vi "UHR-Fleezers Control (host) - 12.2.vi"() -> ()   [LabVIEW 2014] (continued)
                                n838 = flat-sequence {
                                tunnel: [w1198] -> w1193
                                tunnel: w1192 -> [w1198]
                                tunnel: [w1194] -> w1191
                                tunnel: w1190 -> [w1194]
                                tunnel: w1193 -> [w1201]
                                tunnel: w1191 -> [w1199]
                                frame #0 {
                                n839 = local read "Yank Delay (s)"() -> (w1197:dbl)
                                n840 = Multiply(x=w1197, y=1000.0) -> (x*y=w1195:dbl)
                                n841 = Wait (ms)(milliseconds to wait=w1195) -> ()  [unwired: 1 out]
                                }
                                frame #1 {
                                n842 = local read "Yank to which?"() -> (w1200:bool)
                                n843 = case shown="False" w1200 {
                                tunnel: w1201 -> [_ w1229]
                                tunnel: w1199 -> [w1202 _]
                                frame False {
                                n844 = flat-sequence {
                                tunnel: w1202 -> [w1203]
                                frame #0 {
                                n845 = property on="Trap Pos FB SP" class="DigNum (strict)"("Val(Sgnl)"=w1203) -> ()  [unwired: 2 in, 2 out]
                                }
                                frame #1 {
                                n846 = Wait (ms)(milliseconds to wait=u32 700) -> ()  [unwired: 1 out]
                                }
                                frame #2 {
                                n847 = local read "Action (%)"() -> (w1208:dbl)
                                n848 = Absolute Value(x=w1208) -> (abs(x)=w1207:dbl)
                                n849 = Greater?(x=w1207, y=70.0) -> (0:w1205:bool)
                                n850 = property on="Remove Action Offset" class="Bool (strict)"("Val(Sgnl)"=w1205) -> ()  [unwired: 2 in, 2 out]
                                }
                                frame #3 {
                                n851 = for {
                                N: 4 -> [_]
                                n852 = flat-sequence {
                                frame #0 {
                                n853 = Wait (ms)(milliseconds to wait=u32 500) -> ()  [unwired: 1 out]
                                }
                                frame #1 {
                                n854 = local read "Action (%)"() -> (w1214:dbl)
                                n855 = Absolute Value(x=w1214) -> (abs(x)=w1213:dbl)
                                n856 = Greater?(x=w1213, y=70.0) -> (0:w1211:bool)
                                n857 = property on="Remove Action Offset" class="Bool (strict)"("Val(Sgnl)"=w1211) -> ()  [unwired: 2 in, 2 out]
                                }
                                }
                                }
                                }
                                frame #4 {
                                n858 = local read "Shift confocal"() -> (w1219:bool)
                                n859 = local read "Mean"() -> (w1221:dbl)
                                n860 = Greater?(x=w1221, y=11.0) -> (0:w1218:bool)
                                n861 = Not(x=w1218) -> (.not. x?=w1217:bool)
                                n862 = And(x=w1218, y=w1219) -> (x .and. y?=w1216:bool)
                                n863 = And(x=w1217, y=w1219) -> (x .and. y?=w1215:bool)
                                n864 = case shown="True" w1216 {
                                frame False {
                                }
                                frame True {
                                n865 = local read "Confocal Y 2 (V)"() -> (w1225:dbl)
                                n866 = local read "Confocal X 2 (V)"() -> (w1224:dbl)
                                n867 = property on="AO2" class="Slide (strict)"("Val(Sgnl)"=w1224) -> ()  [unwired: 2 in, 2 out]
                                n868 = property on="AO1" class="Slide (strict)"("Val(Sgnl)"=w1225) -> ()  [unwired: 2 in, 2 out]
                                }
                                }
                                n869 = case shown="True" w1215 {
                                frame False {
                                }
                                frame True {
                                n870 = local read "Confocal X 1 (V)"() -> (w1222:dbl)
                                n871 = local read "Confocal Y 1 (V)"() -> (w1223:dbl)
                                n872 = property on="AO1" class="Slide (strict)"("Val(Sgnl)"=w1223) -> ()  [unwired: 2 in, 2 out]
                                n873 = property on="AO2" class="Slide (strict)"("Val(Sgnl)"=w1222) -> ()  [unwired: 2 in, 2 out]
                                }
                                }
                                }
                                frame #5 {
                                n874 = Wait (ms)(milliseconds to wait=u32 1500) -> ()  [unwired: 1 out]
                                }
                                frame #6 {
                                n875 = property on="Rem fb disp offset" class="Bool (strict)"("Val(Sgnl)"=TRUE ("Value (Signaling)")) -> ()  [unwired: 2 in, 2 out]
                                n876 = property on="Remove Offset" class="Bool (strict)"("Val(Sgnl)"=TRUE ("Value (Signaling)")) -> ()  [unwired: 2 in, 2 out]
                                }
                                }
                                }
                                frame True {
                                n877 = flat-sequence {
                                tunnel: w1229 -> [w1230]
                                frame #0 {
                                n878 = property on="Trap D (MHz)" class="DigNum (strict)"("Val(Sgnl)"=w1230) -> ()  [unwired: 2 in, 2 out]
                                }
                                frame #1 {
                                n879 = Wait (ms)(milliseconds to wait=u32 500) -> ()  [unwired: 1 out]
                                }
                                frame #2 {
                                n880 = local read "Shift confocal"() -> (w1236:bool)
                                n881 = local read "Mean"() -> (w1238:dbl)
                                n882 = Greater?(x=w1238, y=11.0) -> (0:w1235:bool)
                                n883 = Not(x=w1235) -> (.not. x?=w1234:bool)
                                n884 = And(x=w1235, y=w1236) -> (x .and. y?=w1233:bool)
                                n885 = And(x=w1234, y=w1236) -> (x .and. y?=w1232:bool)
                                n886 = case shown="True" w1233 {
                                frame False {
                                }
                                frame True {
                                n887 = local read "Confocal Y 2 (V)"() -> (w1242:dbl)
                                n888 = local read "Confocal X 2 (V)"() -> (w1241:dbl)
                                n889 = property on="AO2" class="Slide (strict)"("Val(Sgnl)"=w1241) -> ()  [unwired: 2 in, 2 out]
                                n890 = property on="AO1" class="Slide (strict)"("Val(Sgnl)"=w1242) -> ()  [unwired: 2 in, 2 out]
                                }
                                }
                                n891 = case shown="True" w1232 {
                                frame False {
                                }
                                frame True {
                                n892 = local read "Confocal Y 1 (V)"() -> (w1240:dbl)
                                n893 = local read "Confocal X 1 (V)"() -> (w1239:dbl)
                                n894 = property on="AO2" class="Slide (strict)"("Val(Sgnl)"=w1239) -> ()  [unwired: 2 in, 2 out]
                                n895 = property on="AO1" class="Slide (strict)"("Val(Sgnl)"=w1240) -> ()  [unwired: 2 in, 2 out]
                                }
                                }
                                }
                                }
                                }
                                }
                                }
                                }
                                }
                                }
                                n896 = local read "Messages"() -> (w1187:string)
                                n897 = Subtract(x=w1179, y=w1178) -> (x-y=w1185:dbl)
                                "Duration (s)" <- w1185
                                n898 = Number To Decimal String(number=w1185, width (-)=i16 0) -> (decimal integer string=w1183:string)
                                n899 = Concatenate Strings(w1183, " s fluorescence event." ("string")) -> (w1181:string)
                                n900 = call "Update messages.vi"("Message to add"=w1181, "Old message string"=w1187) -> ("New message string"=w1186:string)
                                n901 = local write "Reset Force"(FALSE ("Reset Force")) -> ()
                                n902 = local write "Waiting"(TRUE ("Waiting")) -> ()
                                n903 = local write "Messages"(w1186) -> ()
                                n904 = local write "Fl. High"(FALSE ("Fl. High")) -> ()
                                n905 = call <vilib>:"Beep.vi"() -> ()  [unwired: 3 in, 9 out]
                                }
                                }
                                n906 = node-c288() -> ()  [unwired: 2 out]
                              }
                              n907 = node-c288(w1155) -> ()  [unwired: 1 out]
                            }
                          }
                        }
                      }
                      n908 = local read "Trap Pos FB SP"() -> (w1063:fxp<+/-,16,1>)
                      n909 = local read "Trap D (MHz)"() -> (w1068:dbl)
                    }
                  }
                }
                frame #1 {
                  n910 = local read "Stop All"() -> (w1252:bool)
                  n911 = local read "Fl. Triggered..."() -> (w1250:bool)
                  n912 = Not(x=w1250) -> (.not. x?=w1251:bool)
                  n913 = Or(x=w1251, y=w1252) -> (x .or. y?=w1249:bool)
                }
              }
              n914 = case shown="True" w838 {
                frame False {
                }
                frame True {
                  n915 = local read "Confocal Y 1 (V)"() -> (w848:dbl)
                  n916 = local read "Confocal X 1 (V)"() -> (w847:dbl)
                  n917 = property on="AO2" class="Slide (strict)"("Val(Sgnl)"=w847) -> ()  [unwired: 2 in, 2 out]
                  n918 = property on="AO1" class="Slide (strict)"("Val(Sgnl)"=w848) -> ()  [unwired: 2 in, 2 out]
                }
              }
              n919 = case shown="True" w838 {
                frame False {
                }
                frame True {
                  w846 = FALSE ("Fl. High")
                  n920 = local write "Waiting"(w846) -> ()
                  n921 = local write "Fl. High"(w846) -> ()
                }
              }
              n922 = node-c288() -> ()  [unwired: 2 out]
            }
            n923 = node-c288(w836) -> ()  [unwired: 1 out]
          }
        }
      }
      event "Stop All": Value Change {
        n924 = event-data() -> ()  [unwired: 7 out]
        n925 = local read "Stop All"() -> (w1257:bool)
      }
    }
    n926 = node-c288() -> ()  [unwired: 2 out]
  }
  n927 = property on="Saved trap pos" class="WFGraph (strict)"("Visible"=TRUE) -> ()  [unwired: 2 in, 2 out]
  n928 = property on="Trap Delta Graph" class="WFGraph (strict)"("Visible"=FALSE) -> ()  [unwired: 2 in, 2 out]
  n929 = local write "Trap pos"(TRUE ("Trap pos")) -> ()
  n930 = node-c288(2 ("Processor")) -> (w137:T26)  [unwired: 3 out]
  n931 = timed-loop "Control parameters (event loop)" {
    tunnel: w51 -> [w1266]
    shift-right: [w1265] -> _
    shift-left: errorcluster {"status"=FALSE, "code"=0, "source"=""} ("error out") -> [w1264]
    tunnel: [w1263] -> _
    timing: w137 -> [_]
    timing-out: [_] -> w136
    tunnel: w111 -> [w1262]
    tunnel: w55 -> [w1261]
    tunnel: w54 -> [w1260]
    tunnel: w53 -> [w1259]
    tunnel: w52 -> [w1258]
    stop <- w1263 stop-if-true
    n932 = node-c288() -> ()  [unwired: 2 out]
    n933 = event shown="[0] \"AI Count (ticks)\", \"Sets to FIFO (Traps)\", \"Save ave N\", \"FPGA Ave.\", \"# Samples/channel\", \"N sets to save\": Value Change" {
      selector: _ -> [_ _ _ _ _ _ _ _ _ _ _ _ _ _ _ _ _ _ _ _ _ _ _ _ _ _ _ _ _ _ _ _ _ _ _ _ _ _ _ _ _ _ _ _ _ _ _ _ _ _ _ _ _ _ _ _ _ _ _ _ _ _ _ _ _ _ _ _ _ _ _ _ _ _ _ _ _ _ _ _]
      dyn-events: _ -> [_ _ _ _ _ _ _ _ _ _ _ _ _ _ _ _ _ _ _ _ _ _ _ _ _ _ _ _ _ _ _ _ _ _ _ _ _ _ _ _ _ _ _ _ _ _ _ _ _ _ _ _ _ _ _ _ _ _ _ _ _ _ _ _ _ _ _ _ _ _ _ _ _ _ _ _ _ _ _ _]
      timeout: _ -> [_ _ _ _ _ _ _ _ _ _ _ _ _ _ _ _ _ _ _ _ _ _ _ _ _ _ _ _ _ _ _ _ _ _ _ _ _ _ _ _ _ _ _ _ _ _ _ _ _ _ _ _ _ _ _ _ _ _ _ _ _ _ _ _ _ _ _ _ _ _ _ _ _ _ _ _ _ _ _ _]
      tunnel: w1266 -> [w1304 _ _ _ w1342 _ w1364 _ _ _ _ w1430 _ _ w1473 w1479 w1484 w1490 w1526 w1553 w1563 _ w1582 w1586 w1597 w1608 w1619 w1636 w1647 w1658 w1685 w1779 w1786 w1824 _ _ w1884 w1888 w1899 w1903 w1907 _ w1915 _ _ _ _ _ _ _ _ _ _ _ _ _ _ _ _ _ w2296 _ w2313 _ w2320 w2338 _ w2345 w2353 w2368 w2379 w2385 _ w2394 _ w2413 _ _ _ w2488]
      tunnel: [w1303 _ _ _ w1332 _ w1363 _ _ w1395 _ w1409 _ _ w1472 w1475 w1481 w1487 w1525 w1551 w1562 _ w1580 _ w1591 w1602 w1613 w1630 w1641 w1652 w1683 w1777 w1784 w1822 _ _ w1882 w1886 w1889 w1901 w1905 _ w1913 _ _ _ _ _ _ _ _ _ _ _ _ _ _ _ _ _ w2294 _ _ _ _ w2335 _ _ _ _ _ _ _ _ _ _ _ _ _ w2486] -> w1265
      tunnel: w1264 -> [w1302 _ _ _ w1341 _ w1362 _ _ w1395 _ w1429 _ _ w1471 w1474 w1480 w1486 w1524 w1552 w1561 _ w1581 w1585 w1596 w1607 w1618 w1635 w1646 w1657 w1684 w1778 w1785 w1823 _ _ w1883 w1887 w1898 w1902 w1906 _ w1914 _ _ _ _ _ _ _ _ _ _ _ _ _ _ _ _ _ w2295 _ w2312 _ w2319 w2337 _ w2344 w2352 w2367 w2378 w2384 _ w2393 _ w2412 _ _ _ w2487]
      tunnel: [_ _ _ _ _ _ _ _ _ w1394 _ _ _ _ _ _ _ _ _ _ _ _ _ _ _ _ _ _ _ _ _ _ _ _ _ _ _ _ _ _ _ _ _ _ _ _ _ _ _ _ _ _ _ _ _ _ _ _ _ _ _ _ _ _ _ _ _ _ _ _ _ _ _ _ _ _ _ _ _ _] -> w1263
      tunnel: [_ _ _ _ _ _ _ "Round T1 X" _ _ _ _ _ _ _ _ _ _ _ _ _ _ _ _ _ _ _ _ _ _ _ _ _ _ _ _ _ _ _ _ _ _ _ _ _ _ _ _ _ _ _ _ _ _ _ _ _ _ _ _ _ _ _ _ _ _ _ _ _ _ _ _ _ _ _ _ _ _ _ _] -> _
      tunnel: [_ _ _ "Adjust Scale\nto Mean" _ _ _ _ _ _ _ _ _ _ _ _ _ _ _ _ _ _ "Test ttrig" _ _ _ _ _ _ _ _ _ _ _ _ _ _ _ _ _ _ _ _ _ _ _ _ _ _ _ "Flush Sample" "Flush Pump 3" "Flush Pump 1" "Clear Volume" _ _ _ _ _ _ _ _ _ _ _ _ _ _ _ _ _ _ _ _ _ _ _ _ _ _] -> _
      tunnel: [_ _ _ _ _ _ _ _ "Round T2 X" _ "Delayed Interlace Start" _ _ _ _ _ _ _ _ _ _ _ _ _ _ _ _ _ _ _ _ _ _ _ _ _ _ _ _ _ _ _ _ _ _ _ _ _ _ _ _ _ _ _ _ _ _ _ _ _ _ _ _ _ _ _ _ _ _ _ _ _ _ _ _ _ _ _ _ _] -> _
      tunnel: w1262 -> [_ _ _ _ _ _ _ _ _ _ _ _ _ _ _ _ _ _ _ _ _ _ _ _ _ _ _ _ _ _ _ _ _ _ _ _ _ _ _ _ _ _ _ _ _ _ w2073 w2091 w2098 w2103 w2109 _ _ w2208 _ _ _ _ _ _ _ _ _ _ _ _ _ _ _ _ _ _ _ _ _ _ _ _ _ _]
      tunnel: w1261 -> [_ _ _ _ _ _ _ _ _ _ _ _ _ _ _ _ _ _ _ _ _ _ _ _ _ _ _ _ _ _ _ _ _ _ _ _ _ _ _ _ _ _ _ _ w1989 _ _ _ _ _ _ w2139 _ _ w2215 _ w2224 _ w2238 _ _ _ _ _ _ _ _ _ _ _ _ _ _ _ _ _ _ _ _ _]
      tunnel: w1260 -> [_ _ _ _ _ _ _ _ _ _ _ _ _ _ _ _ _ _ _ _ _ _ _ _ _ _ _ _ _ _ _ _ _ _ _ _ _ _ _ _ _ _ _ _ _ _ _ _ _ _ _ _ _ _ _ _ _ _ _ _ _ _ _ _ _ _ _ _ _ _ _ _ _ _ _ _ _ _ _ _]
      tunnel: w1259 -> [_ _ _ _ _ _ _ _ _ _ _ _ _ _ _ _ _ _ _ _ _ _ _ _ _ _ _ _ _ _ _ _ _ _ _ _ _ _ _ _ _ _ _ w1926 _ _ _ _ _ _ _ _ w2169 _ _ w2220 _ w2231 _ w2263 _ _ _ _ _ _ _ _ _ _ _ _ _ _ _ _ _ _ _ _]
      tunnel: w1258 -> [_ _ _ _ _ _ _ _ _ _ _ _ _ _ _ _ _ _ _ _ _ _ _ _ _ _ _ _ _ _ _ _ _ _ _ _ _ _ _ _ _ _ _ _ _ _ _ _ _ _ _ _ _ _ _ _ _ _ _ _ _ _ _ _ _ _ _ _ _ _ _ _ _ _ _ _ _ _ _ _]
      event "AI Count (ticks)", "Sets to FIFO (Traps)", "Save ave N", "FPGA Ave.", "# Samples/channel", "N sets to save": Value Change {
        # "So that if 'Save ave N' is updated, the AOD scanning code updates too."
        n934 = event-data() -> ()  [unwired: 6 out]
        n935 = local read "AI Count (ticks)"() -> (w1284:u32)
        n936 = Boolean To (0,1)(Boolean="Sets to FIFO (Traps)") -> (0, 1=w1294:cluster{"Set 1":i16, "Set 2":i16, "Set 3":i16})
        n937 = Cluster To Array(cluster=w1294) -> (array=w1293:i16[])
        n938 = xnode "Read/Write Control"("FPGA VI Reference In"=w1304, "error in"=w1302, "ai count"=w1284, "AI1 Sets to FIFO"="Sets to FIFO (Traps)", "N of AI1 Int Acq Sets"="N Acq Sets (Traps + Fl.)") -> ("error out"=w1303:errorcluster)  [unwired: 1 out]
        n939 = To Unsigned Long Integer(number=w1293) -> (unsigned 32bit integer=w1273:u32[])
        n940 = local read "Scan steps (AOD)"() -> (w1295:u64)
        n941 = Multiply(x=w1284, y="N Acq Sets (Traps + Fl.)") -> (x*y=w1282:u32)
        n942 = Divide(x=40000000.0, y=w1284) -> (x/y=w1276:dbl)
        "AI rate (Hz)" <- w1276
        "Ave. Rate (Hz)" <- w1276
        n943 = Add Array Elements(numeric array=w1273) -> (sum=w1285:u32)
        "Trap Sets" <- w1285
        n944 = Reciprocal(x=w1276) -> (1/x=→"Ave. Period (s)":dbl)
        n945 = property on="Scan steps (AOD)" class="DigNum (strict)"("Val(Sgnl)"=w1295) -> ()  [unwired: 2 in, 2 out]
        n946 = Divide(x=w1276, y="N Acq Sets (Traps + Fl.)") -> (x/y=w1299:dbl)
        "Data Rate (Hz)" <- w1299
        n947 = Reciprocal(x=w1299) -> (1/x=→"Data Period (s)":dbl)
        n948 = local read "Save ave N"() -> (w1298:dbl)
        n949 = Divide(x=w1299, y=w1298) -> (x/y=w1297:dbl)
        "Save Data Rate (Hz)" <- w1297
        n950 = Reciprocal(x=w1297) -> (1/x=→"Save Data Period (s)":dbl)
        n951 = Multiply(x=w1282, y="# Samples/trap") -> (x*y=w1280:u32)
        "Counts/DMA" <- w1280
        n952 = property on="Trap Disp. Downsample" class="DigNum (strict)"("Maximum"="# Samples/trap") -> ()  [unwired: 2 in, 2 out]
        n953 = Multiply(x=w1285, y="# Samples/trap") -> (x*y=w1274:u32)
        "# Samples/channel" <- w1274
        n954 = Multiply(x=w1274, y=u32 8) -> (x*y=→"Trap AI Elements/DMA read":u32)
        n955 = local read "APD Int. Count"() -> (w1281:u32)
        n956 = Multiply(x=w1274, y=u32 3) -> (x*y=→"Trap Pos Elements/DMA read":u32)
        n957 = Divide(x=w1280, y=w1281) -> (x/y=w1271:dbl)
        "APD Samples/FIFO Acq." <- w1271
        n958 = Divide(x=w1280, y=40000000.0) -> (x/y=w1278:dbl)
        "DMA Update Period (s)" <- w1278
        n959 = Multiply(x=2.0, y=w1271) -> (x*y=→"APD Elements/DMA read":dbl)
        n960 = property on="APD Disp. Downsample" class="DigNum (strict)"("Maximum"=w1271) -> ()  [unwired: 2 in, 2 out]
        n961 = local read "N sets to save"() -> (w1291:u32)
        n962 = Multiply(x=w1278, y=w1291) -> (x*y=→"Total Time (s)":dbl)
        "FPGA Averaging" <- FALSE ("FPGA Averaging")
      }
      event "Remove Offset": Value Change {
        n963 = event-data() -> ()  [unwired: 7 out]
        n964 = local write "Remove Offset"(FALSE ("Remove Offset")) -> ()
        n965 = local read "Bead Mean (nm)"() -> (w1306:dbl)
        n966 = local read "Offset (nm)"() -> (w1307:dbl)
        n967 = Add(x=w1306, y=w1307) -> (x+y=w1305:dbl)
        n968 = local write "Offset (nm)"(w1305) -> ()
        n969 = disable-structure shown="Disabled" {
          frame Disabled {
            n970 = local read "Bead Mean (nm)"() -> (w1312:dbl)
            n971 = Add(y=w1312) -> (x=w1311:dbl, x+y=w1310:dbl)
            n972 = Subtract(x=w1312, y=w1311) -> (x-y=w1309:dbl)
            n973 = property on="Bead Separation" class="WFChart (strict)"("YScale.Minimum"=w1309) -> ()  [unwired: 2 in, 2 out]
            n974 = property on="Bead Separation" class="WFChart (strict)"("YScale.Maximum"=w1310) -> ()  [unwired: 2 in, 2 out]
          }
          frame Enabled {
          }
        }
      }
      event "Detector Type": Value Change {
        n975 = event-data() -> ()  [unwired: 7 out]
        n976 = local read "AI labels"() -> (w1313:string[])
        n977 = property on="High Res. Display" class="Ring (strict)"("Strings []"=w1313) -> ()  [unwired: 2 in, 2 out]
        n978 = Build Array (concatenate)(w1313, "none") -> (w1314:string[])
        n979 = property on="FFT 1 Choice 1" class="Ring (strict)"("Strings []"=w1314) -> ()  [unwired: 2 in, 2 out]
        n980 = property on="FFT 1 Choice 2" class="Ring (strict)"("Strings []"=w1314) -> ()  [unwired: 2 in, 2 out]
        n981 = property on="FFT 2 Choice 1" class="Ring (strict)"("Strings []"=w1314) -> ()  [unwired: 2 in, 2 out]
        n982 = property on="FFT 2 Choice 2" class="Ring (strict)"("Strings []"=w1314) -> ()  [unwired: 2 in, 2 out]
        n983 = Bundle("APD 1", "APD 2") -> (w1317:cluster{string, string})  [unwired: 1 out]
        n984 = Cluster To Array(cluster=w1317) -> (array=w1315:string[])
        n985 = Build Array (concatenate)(w1315, w1314) -> (w1319:string[])
        n986 = Array Size(array=w1319) -> (size(s)=w1320:i32)
        n987 = property on="Signals to Plot" class="LstBox (strict)"("Item Names"=w1319) -> ()  [unwired: 2 in, 2 out]
        n988 = property on="Signals to Plot" class="LstBox (strict)"("Number of Rows"=w1320) -> ()  [unwired: 2 in, 2 out]
        n989 = property on="All Signals" class="WFChart (strict)"("LegNumRows"=w1320) -> ()  [unwired: 2 in, 2 out]
      }
      event "Adjust Scale\nto Mean": Value Change {
        n990 = event-data() -> ()  [unwired: 7 out]
        n991 = local read "APD 1 Rate (Hz)"() -> (w1329:dbl)
        n992 = Multiply(x=1000.0, y="Above (kHz)") -> (x*y=w1327:dbl)
        n993 = Multiply(x=1000.0, y="Below (kHz)") -> (x*y=w1325:dbl)
        n994 = Add(x=w1327, y=w1329) -> (x+y=w1322:dbl)
        n995 = Subtract(x=w1329, y=w1325) -> (x-y=w1323:dbl)
        n996 = property on="APD Chart" class="WFChart (strict)"("YScale.Minimum"=w1323) -> ()  [unwired: 2 in, 2 out]
        n997 = property on="APD Chart" class="WFChart (strict)"("YScale.Maximum"=w1322) -> ()  [unwired: 2 in, 2 out]
      }
      event "Phase adj. (AI1)", "+ phase (AI1)", "- phase (AI1)": Value Change {
        n998 = event-data() -> ()  [unwired: 7 out]
        n999 = Negate(x="Phase adj. (AI1)") -> (-x=w1339:i16)
        n1000 = Select(t=w1339, s="- phase (AI1)", f="Phase adj. (AI1)") -> (s? t:f=w1338:i16)
        n1001 = xnode "Read/Write Control"("FPGA VI Reference In"=w1342, "error in"=w1341, "Phase count adjustment"=w1338) -> ("FPGA VI Reference Out"=w1337:T22, "error out"=w1336:errorcluster)
        n1002 = Or(x="- phase (AI1)", y="+ phase (AI1)") -> (x .or. y?=w1333:bool)
        n1003 = xnode "Read/Write Control"("FPGA VI Reference In"=w1337, "error in"=w1336, "+ phase"=w1333) -> ("error out"=w1332:errorcluster)  [unwired: 1 out]
      }
      event "Signals to Plot": Double Click {
        w1345 = u32 9868950 ("Color Box")
        n1004 = event-data() -> ("Row"=w1347:i32)  [unwired: 9 out]
        n1005 = property on="All Signals" class="WFChart (strict)"("Active Plot"=w1347) -> (error out=w1358:errorcluster)  [unwired: 2 in, 1 out]
        n1006 = property on="All Signals" class="WFChart (strict)" props=["Plot", "Visible?", "Plot", "Plot Color"](error in=w1358) -> (error out=w1357:errorcluster, "Plot.Visible?"=w1356:bool)  [unwired: 1 in, 2 out]
        n1007 = Select(t=FALSE ("Plot.Visible"), s=w1356, f=TRUE ("Plot.Visible")) -> (s? t:f=w1351:bool)
        n1008 = property on="All Signals" class="WFChart (strict)"(error in=w1357, "Plot.Visible?"=w1351) -> (error out=w1353:errorcluster)  [unwired: 1 in, 1 out]
        n1009 = property on="All Signals" class="WFChart (strict)"(error in=w1353) -> (error out=w1348:errorcluster, "Plot.Plot Color"=w1352:u32)  [unwired: 1 in, 1 out]
        n1010 = property on="Signals to Plot" class="LstBox (strict)"(error in=w1348, "Active Row"=w1347) -> (error out=w1346:errorcluster)  [unwired: 1 in, 1 out]
        n1011 = Select(t=w1352, s=w1351, f=u32 0) -> (s? t:f=w1349:u32)
        n1012 = property on="Signals to Plot" class="LstBox (strict)"(error in=w1346, "CellFontColor"=w1349, "SelColor"=w1345, "CellBG"=w1345, "CellFontSize"=u32 20 ("Active Row:Cell Font:Size"), "CellFontBold"=TRUE ("Active Row:Cell Font:Bold")) -> ()  [unwired: 1 in, 2 out]
      }
      event "BD 1 Frequency 1 (MHz)", "BD 1 Frequency 2 (MHz)", "BD 1 Frequency 3 (MHz)", "BD 2 Frequency 1 (MHz)", "BD 2 Frequency 2 (MHz)", "BD 2 Frequency 3 (MHz)", "Trap D (MHz)": Value Change {
        n1013 = event-data() -> ("CtlRef"=w1361:refnum<vi>)  [unwired: 6 out]
        n1014 = control-ref of="Trap D (MHz)"() -> (w1360:refnum<vi>)
        n1015 = Equal?(x=w1360, y=w1361) -> (x = y?=w1359:bool)
        n1016 = case shown="False" "Oscillate Set 1" {
          tunnel: w1364 -> [w1384 _]
          tunnel: [w1383 w1387] -> w1363
          tunnel: w1362 -> [w1382 w1387]
          tunnel: w1359 -> [w1367 _]
          frame False {
            n1017 = local read "BD 1 Frequency 2 (MHz)"() -> (w1371:dbl)
            n1018 = local read "BD 1 Frequency 1 (MHz)"() -> (w1369:dbl)
            n1019 = Subtract(x=w1371, y="Trap D (MHz)") -> (x-y=w1368:dbl)
            n1020 = Select(t=w1368, s=w1367, f=w1369) -> (s? t:f=w1366:dbl)
            n1021 = local read "Y RF Frequency Limits (MHz)"() -> (w1372:T17)
            n1022 = local read "X RF Frequency Limits (MHz)"() -> (w1373:T17)
            n1023 = local read "BD 1 Frequency 3 (MHz)"() -> (w1385:dbl)
            n1024 = local write "BD 1 Frequency 1 (MHz)"(w1366) -> ()
            n1025 = local read "BD 2 Frequency 1 (MHz)"() -> (w1376:dbl)
            n1026 = local read "BD 2 Frequency 2 (MHz)"() -> (w1375:dbl)
            n1027 = local read "BD 2 Frequency 3 (MHz)"() -> (w1386:dbl)
            n1028 = call "set RF board frequency - interlace.vi"("Board 2 Frequency Limits"=w1372, "Board 1 Frequency Limits"=w1373, "error in"=w1382, "FPGA VI Reference In"=w1384, "Board 2 Frequency 3 (MHz)"=w1386, "Board 1 Frequency 3 (MHz)"=w1385, "Board 2 Frequency 2 (MHz)"=w1375, "Board 2 Frequency 1 (MHz)"=w1376, "Board 1 Frequency 2 (MHz)"=w1371, "Board 1 Frequency 1  (MHz)"=w1366) -> ("error out"=w1383:errorcluster)  [unwired: 1 out]
            n1029 = Subtract(x=w1376, y=w1375) -> (x-y=w1380:dbl)
            n1030 = Subtract(x=w1366, y=w1371) -> (x-y=w1381:dbl)
            n1031 = Square(x=w1380) -> (x^2=w1378:dbl)
            n1032 = Square(x=w1381) -> (x^2=w1379:dbl)
            n1033 = Add(x=w1379, y=w1378) -> (x+y=w1377:dbl)
            n1034 = Square Root(x=w1377) -> (sqrt(x)=w1374:dbl)
            n1035 = local write "Trap D (MHz)"(w1374) -> ()
            n1036 = property on="Initial D (MHz)" class="DigNum (strict)"("Val(Sgnl)"=w1374) -> ()  [unwired: 2 in, 2 out]
          }
          frame True {
          }
        }
      }
      event "Round T1 X": Value Change {
        n1037 = event-data() -> ()  [unwired: 7 out]
        n1038 = local read "BD 1 Frequency 1 (MHz)"() -> (w1390:dbl)
        n1039 = Round To Nearest(number=w1390) -> (nearest integer value=w1389:dbl)
        n1040 = property on="BD 1 Frequency 1 (MHz)" class="DigNum (strict)"("Val(Sgnl)"=w1389) -> ()  [unwired: 2 in, 2 out]
      }
      event "Round T2 X": Value Change {
        n1041 = event-data() -> ()  [unwired: 7 out]
        n1042 = local read "BD 1 Frequency 2 (MHz)"() -> (w1392:dbl)
        n1043 = Round To Nearest(number=w1392) -> (nearest integer value=w1391:dbl)
        n1044 = property on="BD 1 Frequency 2 (MHz)" class="DigNum (strict)"("Val(Sgnl)"=w1391) -> ()  [unwired: 2 in, 2 out]
      }
      event "Stop All": Value Change {
        n1045 = event-data() -> ()  [unwired: 7 out]
        n1046 = local read "Stop All"() -> (w1394:bool)
      }
      event "Delayed Interlace Start": Value Change {
        n1047 = event-data() -> ()  [unwired: 7 out]
        n1048 = flat-sequence {
          frame #0 {
            n1049 = Multiply(x="Delay to Interlace (s)", y=1000.0) -> (x*y=w1397:dbl)
            n1050 = Wait (ms)(milliseconds to wait=w1397) -> ()  [unwired: 1 out]
          }
          frame #1 {
            n1051 = property on="Laser interlacing mode (all lasers)" class="RadioBtnsControl (strict)"("Val(Sgnl)"=enum32{"Laser ON", "Laser OFF", "Interlace"}."Interlace" ("Value (Signaling)")) -> ()  [unwired: 2 in, 2 out]
          }
        }
      }
      event "BD 1 Amplitude 1 (%)", "BD 1 Amplitude 2 (%)", "BD 1 Amplitude 3 (%)", "BD 2 Amplitude 1 (%)", "BD 2 Amplitude 2 (%)", "BD 2 Amplitude 3 (%)", "Trap 1 ON", "Trap 2 ON", "Trap 3 ON", "Feedback On/Off", "All FB On/Off": Value Change {
        w1421 = i16 1 ("f")
        n1052 = event-data() -> ()  [unwired: 7 out]
        n1053 = local write "Trap 1 (ON/OFF)"("Trap 1 ON") -> ()
        n1054 = local write "Trap 2 (ON/OFF)"("Trap 2 ON") -> ()
        n1055 = Boolean To (0,1)(Boolean="Trap 3 ON") -> (0, 1=w1422:i16)
        n1056 = Boolean To (0,1)(Boolean="Trap 1 ON") -> (0, 1=w1423:i16)
        n1057 = Boolean To (0,1)(Boolean="Trap 2 ON") -> (0, 1=w1424:i16)
        n1058 = Select(t=w1424, s="Trap ON/OFF X or Y Amp?", f=w1421) -> (s? t:f=w1419:i16)
        n1059 = Select(t=w1423, s="Trap ON/OFF X or Y Amp?", f=w1421) -> (s? t:f=w1420:i16)
        n1060 = Select(t=w1422, s="Trap ON/OFF X or Y Amp?", f=w1421) -> (s? t:f=w1418:i16)
        n1061 = Select(t=w1421, s="Trap ON/OFF X or Y Amp?", f=w1424) -> (s? t:f=w1416:i16)
        n1062 = Select(t=w1421, s="Trap ON/OFF X or Y Amp?", f=w1423) -> (s? t:f=w1417:i16)
        n1063 = Select(t=w1421, s="Trap ON/OFF X or Y Amp?", f=w1422) -> (s? t:f=w1415:i16)
        n1064 = And(x="All FB On/Off", y="Feedback On/Off") -> (x .and. y?=w1413:cluster{"Set 1":bool, "Set 2":bool})
        n1065 = local read "BD 1 Amplitude 1 (%)"() -> (w1433:dbl)
        n1066 = local read "BD 1 Amplitude 2 (%)"() -> (w1432:dbl)
        n1067 = local read "BD 1 Amplitude 3 (%)"() -> (w1431:dbl)
        n1068 = Unbundle By Name(w1413) -> ("Set 1"=w1408:bool, "Set 2"=w1405:bool)
        n1069 = local read "Y RF Amplitude Limits (%)"() -> (w1401:T17)
        n1070 = local read "X RF Amplitude Limits (%)"() -> (w1402:T17)
        n1071 = local read "BD 2 Amplitude 1 (%)"() -> (w1434:dbl)
        n1072 = local read "BD 2 Amplitude 2 (%)"() -> (w1435:dbl)
        n1073 = local read "BD 2 Amplitude 3 (%)"() -> (w1436:dbl)
        n1074 = And(x="Trap 2 ON", y=w1405) -> (x .and. y?=w1403:bool)
        n1075 = And(x="Trap 1 ON", y=w1408) -> (x .and. y?=w1406:bool)
        n1076 = Multiply(x=w1420, y=w1433) -> (x*y=w1428:dbl)
        n1077 = Multiply(x=w1432, y=w1419) -> (x*y=w1426:dbl)
        n1078 = Multiply(x=w1431, y=w1418) -> (x*y=w1427:dbl)
        n1079 = Multiply(x=w1434, y=w1417) -> (x*y=w1437:dbl)
        n1080 = Multiply(x=w1435, y=w1416) -> (x*y=w1438:dbl)
        n1081 = Multiply(x=w1436, y=w1415) -> (x*y=w1439:dbl)
        n1082 = call "set RF board amplitude - interlace.vi"("Board 2 Amplitude Limits"=w1401, "Board 1 Amplitude Limits"=w1402, "error in"=w1429, "FPGA VI Reference In"=w1430, "Board 2 Amplitude 3 (%)"=w1439, "Board 1 Amplitude 3 (%)"=w1427, "Board 2 Amplitude 2 (%)"=w1438, "Board 2 Amplitude 1 (%)"=w1437, "Board 1 Amplitude 2 (%)"=w1426, "Board 1 Amplitude 1 (%)"=w1428) -> ("error out"=w1410:errorcluster, "FPGA VI Reference Out"=w1411:T22)
        n1083 = xnode "Read/Write Control"("FPGA VI Reference In"=w1411, "error in"=w1410, "FB On/Off Set 1"=w1406, "FB On/Off Set 2"=w1403) -> ("error out"=w1409:errorcluster)  [unwired: 1 out]
      }
      event "Load parameters": Value Change {
        n1084 = event-data() -> ()  [unwired: 7 out]
        n1085 = property on="Saved AOD Raster Scan Parameter Sets" class="Arr (strict)"() -> ("Index Values"=w1450:u32[])  [unwired: 2 in, 2 out]
        n1086 = Index Array(array=w1450, index=0) -> (element=w1447:u32)
        n1087 = local write "Load parameters"(FALSE ("Load parameters")) -> ()
        n1088 = Index Array(array="Saved AOD Raster Scan Parameter Sets", index=w1447) -> (element=w1446:T31)
        n1089 = Unbundle By Name(w1446) -> ("Scan Range AOD (nm) 2"=w1445:dbl, "Step Size AOD (nm) 2"=w1444:dbl, "Scan Speed AOD (nm/s) 2"=w1443:dbl, "Number of scans (AOD) 2"=w1442:u16)
        n1090 = flat-sequence {
          tunnel: w1445 -> [w1453]
          tunnel: w1444 -> [w1452]
          tunnel: w1443 -> [w1451]
          tunnel: w1442 -> [w1454]
          frame #0 {
            n1091 = local write "Scan Speed (nm/s)"(w1451) -> ()
            n1092 = local write "Scan Range (nm)"(w1453) -> ()
            n1093 = local write "Step Size (nm)"(w1452) -> ()
          }
          frame #1 {
            n1094 = property on="Number of F/B Scans (AOD)" class="DigNum (strict)"("Val(Sgnl)"=w1454) -> ()  [unwired: 2 in, 2 out]
          }
        }
      }
      event "Trap 1 (ON/OFF)", "Trap 2 (ON/OFF)": Value Change {
        n1095 = event-data() -> ()  [unwired: 7 out]
        n1096 = property on="Trap 2 ON" class="Bool (strict)"("Val(Sgnl)"="Trap 2 (ON/OFF)") -> ()  [unwired: 2 in, 2 out]
        n1097 = property on="Trap 1 ON" class="Bool (strict)"("Val(Sgnl)"="Trap 1 (ON/OFF)") -> ()  [unwired: 2 in, 2 out]
      }
      event "DIO count 1 (ticks)", "DIO count 2 (ticks)", "DIO count 3 (ticks)", "Interlace", "Number Interlace Sets", "Not-Interlacing Set": Value Change {
        n1098 = event-data() -> ()  [unwired: 7 out]
        n1099 = local read "DIO count 3 (ticks)"() -> (w1467:u32)
        n1100 = local read "DIO count 1 (ticks)"() -> (w1469:u32)
        n1101 = local read "DIO count 2 (ticks)"() -> (w1468:u32)
        n1102 = To Unsigned Byte Integer(number="Not-Interlacing Set") -> (unsigned 8bit integer=w1458:u8)
        n1103 = Add(x=w1458, y=u8 1) -> (x+y=w1462:u8)
        n1104 = xnode "Read/Write Control"("FPGA VI Reference In"=w1473, "error in"=w1471, "DIO count 1 (ticks)"=w1469, "DIO count 2 (ticks)"=w1468, "DIO count 3 (ticks)"=w1467, "Interlace ON/OFF"="Interlace", "Number Interlace Cycles"="Number Interlace Sets", "Interlace Off Parameters"=w1462) -> ("error out"=w1472:errorcluster)  [unwired: 1 out]
        n1105 = Build Array(w1469, w1468, w1467) -> (w1460:u32[])
        n1106 = Split 1D Array(array=w1460, index="Number Interlace Sets") -> (first subarray=w1470:u32[])  [unwired: 1 out]
        n1107 = Index Array(array=w1460, index=w1458) -> (element=w1459:u32)
        n1108 = Add Array Elements(numeric array=w1470) -> (sum=w1464:u32)
        n1109 = Select(t=w1464, s="Interlace", f=w1459) -> (s? t:f=→"Total Counts (ticks)":u32)
      }
      event "Reset Feedback": Value Change {
        n1110 = event-data() -> ()  [unwired: 7 out]
        n1111 = Unbundle By Name("Reset Feedback") -> ("Set 1"=w1477:bool, "Set 2"=w1476:bool)
        n1112 = xnode "Read/Write Control"("FPGA VI Reference In"=w1479, "error in"=w1474, "FB Reset Set 1"=w1477, "FB Reset Set 2"=w1476) -> ("error out"=w1475:errorcluster)  [unwired: 1 out]
      }
      event "PID Gains": Value Change {
        n1113 = event-data() -> ()  [unwired: 7 out]
        n1114 = Unbundle By Name("PID Gains") -> ("Set 1"=w1483:T15, "Set 2"=w1482:T15)
        n1115 = xnode "Read/Write Control"("FPGA VI Reference In"=w1484, "error in"=w1480, "FB Gains Set 1"=w1483, "FB Gains Set 2"=w1482) -> ("error out"=w1481:errorcluster)  [unwired: 1 out]
      }
      event "AI2 to Setpoint", "Setpoints (V)": Value Change {
        n1116 = event-data() -> ()  [unwired: 7 out]
        n1117 = xnode "Read/Write Control"("FPGA VI Reference In"=w1490, "error in"=w1486) -> ("FPGA VI Reference Out"=w1489:T22, "error out"=w1488:errorcluster, "AI2 Y Sum Set 1"=w1497:i16, "AI2 Y Sum Set 2"=w1496:i16)
        n1118 = Cluster To Array(cluster="AI2 to Setpoint") -> (array=w1500:bool[])
        n1119 = local read "AI2 (V)"() -> (w1498:cluster{"Set 1":dbl, "Set 2":dbl})
        n1120 = Or Array Elements(Boolean array=w1500) -> (logical OR=w1501:bool)
        n1121 = Bundle By Name(cluster=w1498, "Set 1"=w1497, "Set 2"=w1496) -> (w1495:cluster{"Set 1":dbl, "Set 2":dbl})
        n1122 = Divide(x=w1495, y=3276.7) -> (x/y=w1494:cluster{"Set 1":dbl, "Set 2":dbl})
        "AI2 (V)" <- w1494
        n1123 = case shown="True" w1501 {
          tunnel: [w1504 w1521] -> w1493
          tunnel: "AI2 to Setpoint" -> [_ w1517]
          tunnel: "Setpoints (V)" -> [w1505 w1520]
          tunnel: w1494 -> [_ w1514]
          frame False {
            n1124 = Multiply(x=3276.7, y=w1505) -> (x*y=w1506:cluster{"Set 1":dbl, "Set 2":dbl})
            n1125 = To Word Integer(number=w1506) -> (16bit integer=w1504:cluster{"Set 1":i16, "Set 2":i16})
          }
          frame True {
            n1126 = Unbundle By Name(w1514) -> ("Set 1"=w1513:dbl, "Set 2"=w1512:dbl)
            n1127 = Unbundle By Name(w1520) -> ("Set 1"=w1519:dbl, "Set 2"=w1518:dbl)
            n1128 = Unbundle By Name(w1517) -> ("Set 1"=w1516:bool, "Set 2"=w1515:bool)
            n1129 = Select(t=w1513, s=w1516, f=w1519) -> (s? t:f=w1511:dbl)
            n1130 = Select(t=w1512, s=w1515, f=w1518) -> (s? t:f=w1510:dbl)
            n1131 = Bundle By Name(cluster=w1520, "Set 1"=w1511, "Set 2"=w1510) -> (w1508:cluster{"Set 1":dbl, "Set 2":dbl})
            n1132 = local write "Setpoints (V)"(w1508) -> ()
            n1133 = Multiply(x=3276.7, y=w1508) -> (x*y=w1509:cluster{"Set 1":dbl, "Set 2":dbl})
            n1134 = To Word Integer(number=w1509) -> (16bit integer=w1521:cluster{"Set 1":i16, "Set 2":i16})
          }
        }
        n1135 = Unbundle By Name(w1493) -> ("Set 1"=w1492:i16, "Set 2"=w1491:i16)
        n1136 = xnode "Read/Write Control"("FPGA VI Reference In"=w1489, "error in"=w1488, "FB Setpoint Set 1"=w1492, "FB Setpoint Set 2"=w1491) -> ("error out"=w1487:errorcluster)  [unwired: 1 out]
      }
      event "Invert laser interlacing": Value Change {
        n1137 = event-data() -> ()  [unwired: 7 out]
        n1138 = xnode "Read/Write Control"("FPGA VI Reference In"=w1526, "error in"=w1524, "Invert GI"="Invert laser interlacing", "Invert GI 2"="Invert laser interlacing", "Invert RI"="Invert laser interlacing", "Invert RI 2"="Invert laser interlacing") -> ("error out"=w1525:errorcluster)  [unwired: 1 out]
      }
      event "Green FB Setpoint (mV)", "Green FB Gains", "Green FB On/Off", "Green intensity % (FB OFF)", "Green int current ON count adj", "Red intensity % (FB OFF)", "Red FB Gains", "Red FB On/Off", "Red FB Setpoint (mV)": Value Change {
        n1139 = event-data() -> ()  [unwired: 7 out]
        n1140 = local read "Green FB Setpoint (mV)"() -> (w1542:dbl)
        n1141 = local read "Green intensity % (FB OFF)"() -> (w1545:dbl)
        n1142 = local read "Red intensity % (FB OFF)"() -> (w1535:dbl)
        n1143 = local read "Red FB Setpoint (mV)"() -> (w1531:dbl)
        n1144 = Multiply(x=w1531, y=3.2767) -> (x*y=w1529:dbl)
        n1145 = Multiply(x=w1542, y=3.2767) -> (x*y=w1541:dbl)
        n1146 = Multiply(x=w1545, y=655.35) -> (x*y=w1546:dbl)
        n1147 = Multiply(x=w1535, y=655.35) -> (x*y=w1533:dbl)
        n1148 = To Unsigned Word Integer(number=w1546) -> (unsigned 16bit integer=w1544:u16)
        n1149 = To Unsigned Word Integer(number=w1533) -> (unsigned 16bit integer=w1532:u16)
        n1150 = local read "Green int current ON count adj"() -> (w1549:u16)
        n1151 = local read "Green FB Gains"() -> (w1548:T15)
        n1152 = local read "Laser interlacing mode (all lasers)"() -> (w1538:enum32{"Laser ON", "Laser OFF", "Interlace"})
        n1153 = local read "Green ON/Interlacing"() -> (w1539:bool)
        n1154 = local read "Red FB On/Off"() -> (w1528:bool)
        n1155 = local read "Green FB On/Off"() -> (w1550:bool)
        n1156 = local read "Red FB Gains"() -> (w1527:T15)
        n1157 = Equal?(x=w1538, y=enum32{"Laser ON", "Laser OFF", "Interlace"}."Interlace") -> (x = y?=w1536:bool)
        n1158 = Compound Arithmetic op=AND(w1536, w1550, w1539) -> (w1540:bool)
        n1159 = xnode "Read/Write Control"("FPGA VI Reference In"=w1553, "error in"=w1552, "Green FB Setpoint"=w1541, "Green FB On/Off"=w1540, "Current Out"=w1544, "Green int current ON count adj"=w1549, "Green FB Gains"=w1548, "RI Current Out"=w1532, "Red FB Setpoint"=w1529, "Red FB On/Off"=w1528, "Red FB Gains"=w1527) -> ("error out"=w1551:errorcluster)  [unwired: 1 out]
      }
      event "Laser interlacing mode (all lasers)", "Green ON/Interlacing", "Red Laser ON/Interlacing": Value Change {
        n1160 = event-data() -> ()  [unwired: 7 out]
        n1161 = local write "Green Laser ON/OFF"("Green ON/Interlacing") -> ()
        n1162 = case shown="True" "Green ON/Interlacing" {
          tunnel: "Laser interlacing mode (all lasers)" -> [_ w1577]
          tunnel: [enum32{"Laser ON", "Laser OFF", "Interlace"}."Laser OFF" ("Green laser mode") w1577] -> w1560
          tunnel: [FALSE w1573] -> w1559
          frame False {
          }
          frame True {
            n1163 = local read "Green FB On/Off"() -> (w1574:bool)
            n1164 = Equal?(x=w1577, y=enum32{"Laser ON", "Laser OFF", "Interlace"}."Interlace") -> (x = y?=w1575:bool)
            n1165 = And(x=w1575, y=w1574) -> (x .and. y?=w1573:bool)
          }
        }
        n1166 = case shown="True" "Red Laser ON/Interlacing" {
          tunnel: "Laser interlacing mode (all lasers)" -> [_ w1569]
          tunnel: [FALSE w1566] -> w1554
          tunnel: [enum32{"Laser ON", "Laser OFF", "Interlace"}."Laser OFF" ("Green laser mode") w1569] -> w1555
          frame False {
          }
          frame True {
            n1167 = local read "Red FB On/Off"() -> (w1567:bool)
            n1168 = Equal?(x=w1569, y=enum32{"Laser ON", "Laser OFF", "Interlace"}."Interlace") -> (x = y?=w1568:bool)
            n1169 = And(x=w1568, y=w1567) -> (x .and. y?=w1566:bool)
          }
        }
        n1170 = xnode "Read/Write Control"("FPGA VI Reference In"=w1563, "error in"=w1561, "Operating Mode"=w1560, "Operating Mode 2"=w1560, "Green FB On/Off"=w1559, "Red operating mode"=w1555, "RI operating mode 2"=w1555, "Red FB On/Off"=w1554) -> ("error out"=w1562:errorcluster)  [unwired: 1 out]
      }
      event "Green Laser ON/OFF": Value Change {
        n1171 = event-data() -> ()  [unwired: 7 out]
        n1172 = property on="Green ON/Interlacing" class="Bool (strict)"("Val(Sgnl)"="Green Laser ON/OFF") -> ()  [unwired: 2 in, 2 out]
      }
      event "Test ttrig": Value Change {
        n1173 = event-data() -> ()  [unwired: 7 out]
        n1174 = xnode "Read/Write Control"("FPGA VI Reference In"=w1582, "error in"=w1581, "TTrig?"=TRUE) -> ("error out"=w1580:errorcluster)  [unwired: 1 out]
      }
      event "Neg. TTrig FPGA": Value Change {
        n1175 = event-data() -> ()  [unwired: 7 out]
        n1176 = xnode "Read/Write Control"("FPGA VI Reference In"=w1586, "error in"=w1585, "TTrig Negate Pos"="Neg. TTrig FPGA") -> ()  [unwired: 2 out]
      }
      event "- phase (APD 1 Gate)", "+ phase (APD 1 Gate)": Value Change {
        n1177 = event-data() -> ()  [unwired: 7 out]
        n1178 = local read "Phase Adj. (APD 1 Gate)"() -> (w1587:i16)
        n1179 = Negate(x=w1587) -> (-x=w1595:i16)
        n1180 = Select(t=w1595, s="- phase (APD 1 Gate)", f=w1587) -> (s? t:f=w1594:i16)
        n1181 = Or(x="- phase (APD 1 Gate)", y="+ phase (APD 1 Gate)") -> (x .or. y?=w1590:bool)
        n1182 = xnode "Read/Write Control"("FPGA VI Reference In"=w1597, "error in"=w1596, "Phase count adjustment (APD 1 Gate)"=w1594) -> ("FPGA VI Reference Out"=w1592:T22, "error out"=w1593:errorcluster)
        n1183 = xnode "Read/Write Control"("FPGA VI Reference In"=w1592, "error in"=w1593, "+ phase (APD 1 Gate)"=w1590) -> ("error out"=w1591:errorcluster)  [unwired: 1 out]
      }
      event "+ phase (APD 2 Gate)", "- phase (APD 2 Gate)": Value Change {
        n1184 = event-data() -> ()  [unwired: 7 out]
        n1185 = local read "Phase Adj. (APD 2 Gate)"() -> (w1598:i16)
        n1186 = Negate(x=w1598) -> (-x=w1606:i16)
        n1187 = Select(t=w1606, s="- phase (APD 2 Gate)", f=w1598) -> (s? t:f=w1605:i16)
        n1188 = Or(x="- phase (APD 2 Gate)", y="+ phase (APD 2 Gate)") -> (x .or. y?=w1601:bool)
        n1189 = xnode "Read/Write Control"("FPGA VI Reference In"=w1608, "error in"=w1607, "Phase count adjustment (APD 2 Gate)"=w1605) -> ("FPGA VI Reference Out"=w1603:T22, "error out"=w1604:errorcluster)
        n1190 = xnode "Read/Write Control"("FPGA VI Reference In"=w1603, "error in"=w1604, "+ phase (APD 2 Gate)"=w1601) -> ("error out"=w1602:errorcluster)  [unwired: 1 out]
      }
      event "Phase Adj. (APD Acq)", "+ phase (APD Acq)", "- phase (APD Acq)": Value Change {
        n1191 = event-data() -> ()  [unwired: 7 out]
        n1192 = local read "Phase Adj. (APD Acq)"() -> (w1611:i16)
        n1193 = Negate(x=w1611) -> (-x=w1617:i16)
        n1194 = Select(t=w1617, s="+ phase (APD Acq)", f=w1611) -> (s? t:f=w1616:i16)
        n1195 = Or(x="+ phase (APD Acq)", y="- phase (APD Acq)") -> (x .or. y?=w1612:bool)
        n1196 = xnode "Read/Write Control"("FPGA VI Reference In"=w1619, "error in"=w1618, "Phase Count Adjustment (APD Acq)"=w1616) -> ("FPGA VI Reference Out"=w1614:T22, "error out"=w1615:errorcluster)
        n1197 = xnode "Read/Write Control"("FPGA VI Reference In"=w1614, "error in"=w1615, "+ phase (APD Acq)"=w1612) -> ("error out"=w1613:errorcluster)  [unwired: 1 out]
      }
      event "Phase adj. (GI)", "+ phase (GI)", "- phase (GI)", "+phase (RI)", "- phase (RI)", "Phase adj. (RI)": Value Change {
        n1198 = event-data() -> ()  [unwired: 7 out]
        n1199 = Negate(x="Phase adj. (GI)") -> (-x=w1634:i16)
        n1200 = Select(t=w1634, s="+ phase (GI)", f="Phase adj. (GI)") -> (s? t:f=w1633:i16)
        n1201 = Or(x="+ phase (GI)", y="- phase (GI)") -> (x .or. y?=w1629:bool)
        n1202 = Negate(x="Phase adj. (RI)") -> (-x=w1624:i16)
        n1203 = Select(t=w1624, s="+phase (RI)", f="Phase adj. (RI)") -> (s? t:f=w1621:i16)
        n1204 = Or(x="+phase (RI)", y="- phase (RI)") -> (x .or. y?=w1620:bool)
        n1205 = xnode "Read/Write Control"("FPGA VI Reference In"=w1636, "error in"=w1635, "Phase count adjustment (GI)"=w1633, "Phase count adjustment (RI)"=w1621) -> ("FPGA VI Reference Out"=w1631:T22, "error out"=w1632:errorcluster)
        n1206 = xnode "Read/Write Control"("FPGA VI Reference In"=w1631, "error in"=w1632, "+ phase (GI)"=w1629, "+ phase (RI)"=w1620) -> ("error out"=w1630:errorcluster)  [unwired: 1 out]
      }
      event "+ phase (GI) 2", "- phase (GI) 2": Value Change {
        n1207 = event-data() -> ()  [unwired: 7 out]
        n1208 = Negate(x="Phase adj. (GI) 2") -> (-x=w1645:i16)
        n1209 = Select(t=w1645, s="+ phase (GI) 2", f="Phase adj. (GI) 2") -> (s? t:f=w1644:i16)
        n1210 = Or(x="+ phase (GI) 2", y="- phase (GI) 2") -> (x .or. y?=w1640:bool)
        n1211 = xnode "Read/Write Control"("FPGA VI Reference In"=w1647, "error in"=w1646, "Phase count adjustment (GI) 2"=w1644) -> ("FPGA VI Reference Out"=w1642:T22, "error out"=w1643:errorcluster)
        n1212 = xnode "Read/Write Control"("FPGA VI Reference In"=w1642, "error in"=w1643, "+ phase (GI) 2"=w1640) -> ("error out"=w1641:errorcluster)  [unwired: 1 out]
      }
      event "Phase adj. (Green FB)", "- phase (Green FB)", "+ phase (Green FB)": Value Change {
        n1213 = event-data() -> ()  [unwired: 7 out]
        n1214 = Negate(x="Phase adj. (Green FB)") -> (-x=w1656:i16)
        n1215 = Select(t=w1656, s="+ phase (Green FB)", f="Phase adj. (Green FB)") -> (s? t:f=w1655:i16)
        n1216 = Or(x="+ phase (Green FB)", y="- phase (Green FB)") -> (x .or. y?=w1651:bool)
        n1217 = xnode "Read/Write Control"("FPGA VI Reference In"=w1658, "error in"=w1657, "Phase count adjustment (Green FB)"=w1655) -> ("FPGA VI Reference Out"=w1653:T22, "error out"=w1654:errorcluster)
        n1218 = xnode "Read/Write Control"("FPGA VI Reference In"=w1653, "error in"=w1654, "+ phase (Green FB)"=w1651) -> ("error out"=w1652:errorcluster)  [unwired: 1 out]
      }
      event "Invert APD Gate", "APD Gate ON Count", "APD Gate OFF Count", "APD Gate", "APD Integration Time (s)", "APD 1 AO Mult.", "APD 2 AO Mult.", "Duty frequency (ON 1/N cycles)": Value Change {
        n1219 = event-data() -> ()  [unwired: 7 out]
        n1220 = Add(x="Interlace ON count", y="Interlace OFF count") -> (x+y=w1662:u16)
        n1221 = Add(x="APD Gate ON Count", y="APD Gate OFF Count") -> (x+y=w1675:u16)
        n1222 = Multiply(x="Duty frequency (ON 1/N cycles)", y=w1662) -> (x*y=w1661:u16)
        "Green FB Count" <- w1661
        n1223 = Subtract(x=w1661, y="Interlace ON count") -> (x-y=w1659:u16)
        n1224 = Multiply(x=w1675, y="Duty frequency (ON 1/N cycles)") -> (x*y=w1674:u16)
        n1225 = Subtract(x=w1674, y="APD Gate ON Count") -> (x-y=w1673:u16)
        n1226 = local read "DMA Update Period (s)"() -> (w1676:dbl)
        n1227 = Multiply(x="APD Integration Time (s)", y=40000000.0) -> (x*y=w1681:dbl)
        n1228 = Reciprocal(x="APD Integration Time (s)") -> (1/x=→"APD Acq Rate (Hz)":dbl)
        n1229 = To Unsigned Long Integer(number=w1681) -> (unsigned 32bit integer=w1665:u32)
        "APD Int. Count" <- w1665
        n1230 = xnode "Read/Write Control"("FPGA VI Reference In"=w1685, "error in"=w1684, "Invert APD Gate"="Invert APD Gate", "APD Gate ON Count"="APD Gate ON Count", "APD Gate OFF Count"=w1673, "APD Acq Rate Count"=w1665, "APD Gate Operating Mode"="APD Gate", "APD 1 AO scale factor"="APD 1 AO Mult.", "APD 2 AO scale factor"="APD 2 AO Mult.", "Green interlace ON count"="Interlace ON count", "Green interlace OFF count"=w1659, "Green interlace ON count 2"="Interlace ON count", "Green interlace OFF count 2"=w1659, "Green FB Count"=w1661, "RI ON count"="Interlace ON count", "RI OFF count"=w1659) -> ("error out"=w1683:errorcluster)  [unwired: 1 out]
        n1231 = Divide(x=w1676, y="APD Integration Time (s)") -> (x/y=w1679:dbl)
        n1232 = Multiply(x=2.0, y=w1679) -> (x*y=w1678:dbl)
        n1233 = local write "APD Samples/FIFO Acq."(w1679) -> ()
        n1234 = local write "APD Elements/DMA read"(w1678) -> ()
      }
      event "Number of F/B Scans (AOD)", "Scan Speed (nm/s)", "Scan BD", "Initial D (MHz)", "Step Size (nm)", "Scan Range (nm)", "Wiggle amp 1 (units?)": Value Change {
        w1747 = 123.0  # AOM cal (nm/MHz)
        n1235 = event-data() -> ()  [unwired: 7 out]
        n1236 = local read "BD 1 Frequency 1 (MHz)"() -> (w1730:dbl)
        n1237 = local read "AOM X Cal (nm/MHz)"() -> (w1722:dbl)
        n1238 = local read "BD 2 Frequency 1 (MHz)"() -> (w1736:dbl)
        n1239 = local read "X RF Frequency Limits (MHz)"() -> (w1734:T17)
        n1240 = local read "Y RF Frequency Limits (MHz)"() -> (w1731:T17)
        n1241 = Negate(x="Scan Range (nm)") -> (-x=w1700:dbl)
        n1242 = Divide(x=w1700, y=w1722) -> (x/y=w1704:dbl)
        n1243 = Select(t=w1734, s="Scan BD", f=w1731) -> (s? t:f=w1733:T17)
        n1244 = Select(t=w1730, s="Scan BD", f=w1736) -> (s? t:f=w1735:dbl)
        n1245 = Unbundle By Name(w1733) -> ("Maximum"=w1742:dbl, "Minimum"=w1741:dbl)
        n1246 = Add(x=w1704, y=w1735) -> (x+y=w1739:dbl)
        n1247 = Divide(x=w1700, y="Step Size (nm)") -> (x/y=w1719:dbl)
        n1248 = Divide(x="Step Size (nm)", y=w1722) -> (x/y=w1728:dbl)
        n1249 = Absolute Value(x=w1719) -> (abs(x)=w1703:dbl)
        n1250 = Sign(1:w1700) -> (0:w1701:dbl)
        n1251 = In Range and Coerce(upper limit=w1742, x=w1739, lower limit=w1741) -> (coerced(x)=w1738:dbl, In Range?=w1740:bool)
        n1252 = To Unsigned Quad Integer(1:w1703) -> (0:w1718:u64)
        "Scan steps (AOD)" <- w1718
        n1253 = call "IR AOM freq to word.vi"("Frequency In (MHz)"=w1728) -> ("Frequency Word Out (double)"=w1725:dbl)
        n1254 = Multiply(x=w1701, y=w1725) -> (x*y=w1702:dbl)
        n1255 = Subtract(x=w1739, y=w1738) -> (x-y=w1737:dbl)
        n1256 = To Quad Integer(1:w1702) -> (0:w1724:i64)
        "Incr. int (AOD)" <- w1724
        n1257 = Subtract(x=w1704, y=w1737) -> (x-y=w1723:dbl)
        "Scan Range (MHz)" <- w1723
        n1258 = Select(t=w1704, s=w1740, f=w1723) -> (s? t:f=w1743:dbl)
        n1259 = Multiply(x=w1723, y=w1722) -> (x*y=w1721:dbl)
        n1260 = Decrement(x=w1718) -> (x-1=w1771:u64)
        n1261 = Negate(x=w1721) -> (-x=w1717:dbl)
        n1262 = local write "Scan Range (nm)"(w1717) -> ()
        n1263 = Divide(x=w1743, y=w1771) -> (x/y=w1727:dbl)
        "Scan Increment (MHz)" <- w1727
        n1264 = call "IR AOM freq to word.vi"("Frequency In (MHz)"=w1727) -> ("Frequency Word Out (double)"=w1726:dbl)
        n1265 = Divide(x="Step Size (nm)", y="Scan Speed (nm/s)") -> (x/y=w1714:dbl)
        n1266 = To Quad Integer(1:w1726) -> ()  [unwired: 1 out]
        n1267 = local read "Number Interlace Sets"() -> (w1698:u8)
        n1268 = local read "AI Count (ticks)"() -> (w1699:u32)
        n1269 = local read "Total Counts (ticks)"() -> (w1697:u32)
        n1270 = local read "# Samples/trap"() -> (w1729:u32)
        n1271 = Multiply(x=w1699, y=w1698) -> (x*y=w1696:u32)
        n1272 = Divide(x=w1697, y=w1696) -> (x/y=w1695:dbl)
        n1273 = Select(t=w1730, s="Scan BD", f=w1736) -> (s? t:f=w1768:dbl)
        "Initial freq. (MHz)" <- w1768
        n1274 = Add(x=w1743, y=w1768) -> (x+y=→"Final freq. (MHz)":dbl)
        n1275 = Divide(x=w1697, y=40000000.0) -> (x/y=w1713:dbl)
        n1276 = Divide(x=w1714, y=w1713) -> (x/y=w1712:dbl)
        n1277 = To Unsigned Quad Integer(1:w1712) -> (0:w1687:u64)
        n1278 = Quotient & Remainder(x=w1687, y=u64 2) -> (x-y*floor(x/y)=w1691:u64)  [unwired: 1 out]
        n1279 = Equal?(x=w1691, y=u64 0) -> (x = y?=w1689:bool)
        n1280 = Decrement(x=w1687) -> (x-1=w1688:u64)
        n1281 = Select(t=w1687, s=w1689, f=w1688) -> (s? t:f=w1686:u64)
        "Cycles/step (AOD)" <- w1686
        n1282 = xnode "Read/Write Control"("FPGA VI Reference In"=w1779, "error in"=w1778, "Scan steps"=w1718, "Number of scans"="Number of F/B Scans (AOD)", "Cycles per step"=w1686, "Scan freq.  increment"=w1724, "Scan BD"="Scan BD") -> ("error out"=w1777:errorcluster)  [unwired: 1 out]
        n1283 = Multiply(x=w1718, y=w1686) -> (x*y=w1772:u64)
        n1284 = Multiply(x=w1772, y=u64 2) -> (x*y=w1694:u64)
        n1285 = Multiply(x=w1695, y=w1694) -> (x*y=w1693:dbl)
        "Data points/scan (f/b)" <- w1693
        n1286 = Multiply(x=w1693, y="Number of F/B Scans (AOD)") -> (x*y=w1775:dbl)
        "Data points/scans" <- w1775
        n1287 = Divide(x=w1775, y=w1729) -> (x/y=→"N sets should be saved":dbl)
        n1288 = Multiply(x=w1772, y=w1713) -> (x*y=w1711:dbl)
        "Time/Scan (s) (AOD)" <- w1711
        n1289 = Select(t=w1743, s="Scan BD", f=0.0) -> (s? t:f=w1769:dbl)
        n1290 = Select(t=0.0, s="Scan BD", f=w1743) -> (s? t:f=w1765:dbl)
        n1291 = local read "BD 2 Frequency 2 (MHz)"() -> (w1761:dbl)
        n1292 = local read "BD 1 Frequency 2 (MHz)"() -> (w1764:dbl)
        n1293 = Add(x=w1765, y=w1736) -> (x+y=w1762:dbl)
        n1294 = Add(x=w1730, y=w1769) -> (x+y=w1763:dbl)
        n1295 = Multiply(x=w1711, y=2.0) -> (x*y=w1710:dbl)
        n1296 = Multiply(x=w1710, y="Number of F/B Scans (AOD)") -> (x*y=w1707:dbl)
        n1297 = Divide(x=w1707, y=60.0) -> (x/y=→"Time to Finish All (min)":dbl)
        n1298 = Add(x="Trap 2 Bead Size (nm)", y="Trap 1 Bead Size (nm)") -> (x+y=w1751:dbl)
        n1299 = Divide(x=w1751, y=2.0) -> (x/y=w1745:dbl)
        n1300 = Subtract(x=w1762, y=w1761) -> (x-y=w1759:dbl)
        n1301 = Subtract(x=w1763, y=w1764) -> (x-y=w1760:dbl)
        n1302 = local read "Initial D (MHz)"() -> (w1748:dbl)
        n1303 = Square(x=w1759) -> (x^2=w1758:dbl)
        n1304 = Square(x=w1760) -> (x^2=w1757:dbl)
        n1305 = Add(x=w1757, y=w1758) -> (x+y=w1756:dbl)
        n1306 = Square Root(x=w1756) -> (sqrt(x)=w1755:dbl)